vi "AeroQuadConfigurator.vi"() -> ()   [LabVIEW 2010] (continued)
              n282 = call "NextState.vi"("Data"=w567, "State"="Read", "Queue In"=w568) -> ()  [unwired: 7 in, 2 out]
            }
          }
          n283 = case shown="Error" w562 {
            selector: w562 -> [w578 w585]
            tunnel: [w578 w583] -> w563
            tunnel: w561 -> [_ _]
            tunnel: w558 -> [_ w588]
            tunnel: [TRUE ("Time has Elapsed") w587] -> w555
            tunnel: w556 -> [_ w584]
            tunnel: w550 -> [w576 _]
            tunnel: w553 -> [w574 _]
            frame No Error {
              n284 = Fract/Exp String To Number(string=w576) -> (number=w573:dbl)  [unwired: 3 in, 1 out]
              n285 = Greater Or Equal?(x=w573, y=w574) -> (x >= y?=w575:bool)
              n286 = case shown="False" w575 {
                tunnel: w573 -> [w580 _]
                tunnel: w574 -> [w579 _]
                frame False {
                  n287 = Format Into String(format string="To use all the features of this version of the Configurator, you must use Flight Software v.%.1f or greater.  The current detected Flight Software version is v.%.1f.", w579, w580) -> (resulting string=w582:string)  [unwired: 2 in, 1 out]
                  n288 = One Button Dialog(message=w582) -> ()  [unwired: 1 in, 1 out]
                }
                frame True {
                }
              }
            }
            frame Error {
              n289 = call "Elapsed Time"("Time Target (s)"=w588, "Reset"=w584) -> ("Time has Elapsed"=w587:bool, "error out"=w586:errorcluster)  [unwired: 10 in, 6 out]
              n290 = Select(t=w585, s=w587, f=w586) -> (s? t:f=w583:errorcluster)
            }
          }
        }
        n291 = Bundle By Name(cluster=w545, "Error"=w539) -> (w544:T2)
      }
      frame "Connect" {
        n292 = Unbundle By Name(w596) -> ("Logger"=w591:bool, "DebugLogger"=w595:refnum<queue>)  [unwired: 1 out]
        n293 = Unbundle By Name(w596) -> ("COM Port"=w606:refnum<visa-resource-name>, "StopTelem"=w594:string, "Version"=w593:string)
        n294 = VISA Write(VISA resource name=w606, write buffer=w594) -> (VISA resource name out=w603:refnum<visa-resource-name>, error out=w602:errorcluster)  [unwired: 1 in, 1 out]
        n295 = call "Time Delay8"("error in (no error)"=w602) -> ("error out"=w601:errorcluster)  [unwired: 10 in]
        n296 = VISA Flush I/O Buffer(VISA resource name=w603, error in (no error)=w601) -> (VISA resource name out=w604:refnum<visa-resource-name>, error out=w605:errorcluster)  [unwired: 1 in]
        n297 = VISA Write(VISA resource name=w604, write buffer=w593, error in (no error)=w605) -> (VISA resource name out=w612:refnum<visa-resource-name>, error out=w611:errorcluster)  [unwired: 1 out]
        n298 = VISA Read(VISA resource name=w612, byte count=u32 1024, error in (no error)=w611) -> (VISA resource name out=w609:refnum<visa-resource-name>, read buffer=w592:string, error out=w610:errorcluster)  [unwired: 1 out]
        n299 = case shown="True" w591 {
          selector: w591 -> [_ w625]
          tunnel: w595 -> [w623 w633]
          tunnel: w594 -> [_ w632]
          tunnel: w593 -> [_ w629]
          tunnel: w592 -> [_ w626]
          tunnel: [_ w625] -> w590
          tunnel: [w623 w624] -> w589
          frame False {
          }
          frame True {
            n300 = call "NextState.vi"("Data"=w632, "State"="Write", "Queue In"=w633) -> ("Queue Out"=w630:refnum<queue>)  [unwired: 7 in, 1 out]
            n301 = call "NextState.vi"("Data"=w629, "State"="Write", "Queue In"=w630) -> ("Queue Out"=w627:refnum<queue>)  [unwired: 7 in, 1 out]
            n302 = call "NextState.vi"("Data"=w626, "State"="Read", "Queue In"=w627) -> ("Queue Out"=w624:refnum<queue>)  [unwired: 7 in, 1 out]
          }
        }
        n303 = Decimal String To Number(string=w592) -> (number=w607:i32)  [unwired: 2 in, 1 out]
        n304 = local read "*Timeout (sec)"() -> (w598:dbl)
        n305 = for {
          N: w607 -> [_]
          tunnel: w609 -> [w647]
          shift-right: [w644] -> w619
          shift-left: w610 -> [w645]
          tunnel: [w641] -> w617 mode=indexing
          tunnel: [w640] -> w616 mode=indexing
          tunnel: [w639] -> w613 mode=indexing
          tunnel: [w638] -> w600
          tunnel: w590 -> [w637]
          tunnel: w589 -> [w636]
          n306 = VISA Read(VISA resource name=w647, byte count=u32 1024, error in (no error)=w645) -> (VISA resource name out=w638:refnum<visa-resource-name>, read buffer=w635:string, error out=w644:errorcluster)  [unwired: 1 out]
          n307 = Match Pattern(string=w635, regular expression=":") -> (before substring=w641:string, after substring=w642:string)  [unwired: 1 in, 2 out]
          n308 = case shown="True" w637 {
            tunnel: w636 -> [_ w650]
            tunnel: w635 -> [_ w648]
            frame False {
            }
            frame True {
              n309 = call "NextState.vi"("Data"=w648, "State"="Read", "Queue In"=w650) -> ()  [unwired: 7 in, 2 out]
            }
          }
          n310 = call <vilib>:"Trim Whitespace.vi"("string"=w642) -> ("trimmed string"=w640:string)  [unwired: 1 in]
          n311 = Build Array(w641, w640) -> (w639:string[])
        }
        n312 = Multiply(x=w598, y=1000.0) -> (x*y=w599:dbl)
        n313 = property class="Instr"(reference=w600, "General Settings:Timeout Value"=w599) -> ()  [unwired: 1 in, 2 out]
        n314 = Unbundle By Name(w619) -> ("status"=w618:bool)
        n315 = property on="Sensors" class="Tbl (strict)"("Row Headers[]"=w617) -> ()  [unwired: 2 in, 2 out]
        n316 = Build Array(w616) -> (w615:string[][])
        n317 = Not(x=w618) -> (.not. x?=w620:bool)
        n318 = case shown="True" w620 {
          tunnel: w621 -> [_ w657]
          frame False {
          }
          frame True {
            n319 = call "NextStates.vi"("States"=string[] ["Update Parameters", "Unlock Controls", "Save Comm Controls", "Lock Comm Controls", "Unlock User Controls"], "Queue In"=w657) -> ("Queue Out"=w653:refnum<queue>)  [unwired: 8 in, 1 out]
            n320 = call "NextState.vi"("Data"="Connected to the AeroQuad!", "State"="Status", "Queue In"=w653) -> ("Queue Out"=w652:refnum<queue>)  [unwired: 7 in, 1 out]
            n321 = call <vilib>:"Beep.vi"() -> ()  [unwired: 12 in]
            n322 = call "NextState.vi"("State"="Load SubPanel", "Queue In"=w652) -> ()  [unwired: 8 in, 2 out]
          }
        }
        n323 = Transpose 2D Array(2D array=w615) -> (transposed array=→"Sensors":string[][])
        n324 = Bundle By Name(cluster=w596, "Config"=w613, "Connected"=w620, "Error"=w619) -> (w622:T2)
      }
      frame "Request Telemetry", "Send Command" {
        # "In a telemetry query, a command will be sent\nfirst, then a telemetry request."
        n325 = Unbundle By Name(w669) -> ("Logger"=w658:bool, "DebugLogger"=w659:refnum<queue>, "oldTelem"=w660:string, "Connected"=w666:bool, "COM Port"=w670:refnum<visa-resource-name>)
        n326 = case shown="True" w666 {
          tunnel: w670 -> [_ w679]
          tunnel: w667 -> [_ w681]
          tunnel: [_ w680] -> w665
          tunnel: w664 -> [w671 _]
          tunnel: w663 -> [w673 _]
          tunnel: [_ w675] -> w662
          tunnel: [_ w678] -> w661
          tunnel: w660 -> [_ w678]
          tunnel: w659 -> [_ w676]
          tunnel: w658 -> [_ w677]
          frame False {
            n327 = Flush Queue(queue=w671) -> (queue out=w672:refnum<queue>)  [unwired: 1 in, 2 out]
            n328 = case shown="\"Send Command\"" w673 {
              tunnel: w672 -> [_ _]
              frame Default {
              }
              frame "Send Command" {
                n329 = One Button Dialog(message="The AeroQuad is not connected to the Configurator!\nErroneous messages may appear.") -> ()  [unwired: 1 in, 1 out]
              }
            }
          }
          frame True {
            n330 = Variant To Data(Variant=w681, type="") -> (data=w675:string)  [unwired: 1 in, 1 out]
            n331 = VISA Write(VISA resource name=w679, write buffer=w675) -> (error out=w680:errorcluster)  [unwired: 1 in, 2 out]
            n332 = case shown="True" w677 {
              tunnel: w676 -> [_ w685]
              tunnel: w675 -> [_ w683]
              frame False {
              }
              frame True {
                n333 = call "NextState.vi"("Data"=w683, "State"="Write", "Queue In"=w685) -> ()  [unwired: 7 in, 2 out]
              }
            }
          }
        }
        n334 = Bundle By Name(cluster=w669, "oldCmd"=w661, "oldTelem"=w662, "Error"=w665) -> (w668:T2)
      }
      frame "Clear Serial Comm" {
        n335 = Unbundle By Name(w692) -> ("Logger"=w687:bool, "DebugLogger"=w686:refnum<queue>, "Connected"=w690:bool, "COM Port"=w693:refnum<visa-resource-name>, "StopTelem"=w688:string)
        n336 = case shown="True" w690 {
          tunnel: w693 -> [_ w704]
          tunnel: [_ w701] -> w689
          tunnel: w688 -> [_ w694]
          tunnel: w687 -> [_ w696]
          tunnel: w686 -> [_ w695]
          frame False {
          }
          frame True {
            n337 = case shown="True" w696 {
              tunnel: w695 -> [_ w709]
              tunnel: w694 -> [_ w708]
              tunnel: w694 -> [_ w705]
              frame False {
              }
              frame True {
                w706 = "Write" ("State")
                n338 = call "NextState.vi"("Data"=w708, "State"=w706, "Queue In"=w709) -> ("Queue Out"=w707:refnum<queue>)  [unwired: 7 in, 1 out]
                n339 = disable-structure shown="Disabled" {
                  disable-tunnel: w707 -> [w712 _]
                  disable-tunnel: w706 -> [w711 _]
                  disable-tunnel: w705 -> [w710 _]
                  frame Disabled {
                    n340 = call "NextState.vi"("Data"=w710, "State"=w711, "Queue In"=w712) -> ()  [unwired: 7 in, 2 out]
                  }
                  frame Enabled {
                  }
                }
              }
            }
            n341 = VISA Write(VISA resource name=w704, write buffer=w694) -> (VISA resource name out=w699:refnum<visa-resource-name>, error out=w702:errorcluster)  [unwired: 1 in, 1 out]
            n342 = call "Time Delay3"("error in (no error)"=w702, "Delay Time (s)"=0.25) -> ("error out"=w698:errorcluster)  [unwired: 9 in]
            n343 = VISA Flush I/O Buffer(VISA resource name=w699, error in (no error)=w698) -> (VISA resource name out=w700:refnum<visa-resource-name>, error out=w697:errorcluster)  [unwired: 1 in]
            n344 = disable-structure shown="Enabled" {
              disable-tunnel: [w720 w721] -> w701
              disable-tunnel: w694 -> [w719 _]
              disable-tunnel: w700 -> [w714 _]
              disable-tunnel: w697 -> [w713 w721]
              frame Disabled {
                n345 = VISA Write(VISA resource name=w714, write buffer=w719, error in (no error)=w713) -> (VISA resource name out=w715:refnum<visa-resource-name>, error out=w717:errorcluster)  [unwired: 1 out]
                n346 = call "Time Delay5"("error in (no error)"=w717, "Delay Time (s)"=0.25) -> ("error out"=w716:errorcluster)  [unwired: 9 in]
                n347 = VISA Flush I/O Buffer(VISA resource name=w715, error in (no error)=w716) -> (error out=w720:errorcluster)  [unwired: 1 in, 1 out]
              }
              frame Enabled {
              }
            }
          }
        }
        n348 = Bundle By Name(cluster=w692, "Error"=w689) -> (w691:T2)
      }
      frame "Reconnect" {
        n349 = in-place {
          in-place-border: [w732] -> w724
          n350 = in-place-cluster #3(w727) -> ("Error"=w734:errorcluster)
          n351 = call "ReconnectDialog.vi"("error in"=w734) -> ("error out"=w733:errorcluster, "AbortConnection"=w732:bool)  [unwired: 9 in]
          n352 = in-place-cluster #3("Error"=w733) -> (w726:T2)
        }
        n353 = case shown="False" w724 {
          tunnel: w725 -> [w729 w731]
          tunnel: [w729 w731] -> w723
          tunnel: ["Open Port" "Unlock User Controls"] -> w722
          frame False {
          }
          frame True {
          }
        }
        n354 = call "NextState.vi"("State"=w722, "Queue In"=w723) -> ()  [unwired: 8 in, 2 out]
      }
      frame "Disconnect" {
        n355 = property on="Load SubPanel" class="Ring (strict)"() -> ("Strings []"=w744:string[], "Value"=w745:i32)  [unwired: 2 in, 2 out]
        n356 = Unbundle By Name(w758) -> ("ConnType"=w741:string, "ModemQueue"=w736:refnum<queue>, "COM Port"=w748:refnum<visa-resource-name>, "StopTelem"=w746:string)
        n357 = Index Array(array=w744, index=w745) -> (element=w743:string)
        n358 = call "NextState.vi"("State"="Lock Controls", "Queue In"=w754) -> ("Queue Out"=w752:refnum<queue>)  [unwired: 8 in, 1 out]
        n359 = VISA Write(VISA resource name=w748, write buffer=w746) -> (VISA resource name out=w747:refnum<visa-resource-name>)  [unwired: 1 in, 2 out]
        n360 = VISA Close(VISA resource name=w747) -> ()  [unwired: 1 in, 1 out]
        n361 = call "PriorityState.vi"("Data"="Disconnected from AeroQuad", "State"="Status", "Queue In"=w752) -> ("Queue Out"=w751:refnum<queue>)  [unwired: 7 in, 1 out]
        n362 = Equal?(x="Modem Telemetry Initialize", y=w741) -> (x = y?=w738:bool)
        n363 = Equal?(x="Waypoint Configuration", y=w743) -> (x = y?=w739:bool)
        n364 = Compound Arithmetic op=AND(w739, w738) -> (w737:bool)
        n365 = call "NextState.vi"("State"="Unlock Comm Controls", "Queue In"=w751) -> ("Queue Out"=w735:refnum<queue>)  [unwired: 8 in, 1 out]
        n366 = case shown="True" w737 {
          tunnel: w736 -> [_ w768]
          tunnel: w735 -> [w760 w770]
          frame False {
            n367 = call "NextState.vi"("State"="Unlock User Controls", "Queue In"=w760) -> ()  [unwired: 8 in, 2 out]
          }
          frame True {
            n368 = Flush Queue(queue=w768) -> (queue out=w767:refnum<queue>)  [unwired: 1 in, 2 out]
            n369 = Enqueue Element(queue=w767, element="***Disconnect***") -> (error out=w766:errorcluster)  [unwired: 2 in, 2 out]
            n370 = call "NextState.vi"("Error In"=w766, "State"="Lock User Controls", "Queue In"=w770) -> ("Queue Out"=w765:refnum<queue>)  [unwired: 7 in, 1 out]
            n371 = call "NextState.vi"("Data"="Disconnected from AeroQuad" ("State"), "State"="Status", "Queue In"=w765) -> ("Queue Out"=w762:refnum<queue>)  [unwired: 7 in, 1 out]
            n372 = call "NextState.vi"("State"="Clear Queue", "Queue In"=w762) -> ()  [unwired: 8 in, 2 out]
          }
        }
        n373 = Bundle By Name(cluster=w758, "Connected"=FALSE) -> (w757:T2)
      }
      frame "Update Timeout" {
        n374 = Unbundle By Name(w772) -> ("COM Port"=w776:refnum<visa-resource-name>)
        n375 = Variant To Data(Variant=w775, type=u32 0 ("General Settings:Timeout Value")) -> (data=w773:u32)  [unwired: 1 in, 1 out]
        n376 = property class="Instr"(reference=w776, "Timeout"=w773) -> ()  [unwired: 1 in, 2 out]
      }
      frame "Default Timeout" {
        n377 = Unbundle By Name(w781) -> ("COM Port"=w782:refnum<visa-resource-name>)
        n378 = local read "*Timeout (sec)"() -> (w778:dbl)
        n379 = Compound Arithmetic op=MULTIPLY(w778, 1000.0 ("value")) -> (w780:dbl)
        n380 = To Unsigned Long Integer(number=w780) -> (unsigned 32bit integer=w777:u32)
        n381 = property class="Instr"(reference=w782, "Timeout"=w777) -> ()  [unwired: 1 in, 2 out]
      }
      frame "Connection Type" {
        n382 = Variant To Data(Variant=w785, type="") -> (data=w783:string)  [unwired: 1 in, 1 out]
        n383 = case shown="\"Modem\"" w783 {
          tunnel: w789 -> [w791 w797]
          tunnel: ["Modem Telemetry Initialize" "Check Connection"] -> w786
          frame "Modem" {
            w795 = 3 items=["Initial Setup", "3-D View", "Vehicle Status", "Waypoint Configuration", "Motor Commands", "Serial Monitor", "Vehicle Attitude", "Sensor Data", "Transmitter Data"] ("Load SubPanel")
            n384 = call "NextState.vi"("State"="Lock User Controls", "Queue In"=w791) -> ("Queue Out"=w790:refnum<queue>)  [unwired: 8 in, 1 out]
            n385 = local write "Load SubPanel"(w795) -> ()
            n386 = local write "*Baud Rate"("1200" ("*Baud Rate")) -> ()
            n387 = call "NextState.vi"("State"="Load SubPanel", "Queue In"=w790) -> ()  [unwired: 8 in, 2 out]
          }
          frame "USB/XBee", Default {
            n388 = call "NextState.vi"("State"="Unlock User Controls", "Queue In"=w797) -> ()  [unwired: 8 in, 2 out]
            n389 = property on="Load SubPanel" class="Ring (strict)"("DisabledEnum"=T3."Enabled" ("Disabled")) -> ()  [unwired: 2 in, 2 out]
          }
        }
        n390 = Bundle By Name(cluster=w788, "ConnType"=w786) -> (w787:T2)
      }
      frame "Modem Telemetry Initialize" {
        # "Modem queue initialized in \"Load SubPanels\" state for convenience."
        n391 = Unbundle By Name(w807) -> ("ModemQueue"=w803:refnum<queue>)
        n392 = call "NextState.vi"("State"="Unlock Controls", "Queue In"=w815) -> ("Queue Out"=w811:refnum<queue>)  [unwired: 8 in, 1 out]
        n393 = Lossy Enqueue Element(queue=w803, element="Move Slider Modem" ("State")) -> (queue out=w801:refnum<queue>)  [unwired: 1 in, 3 out]
        n394 = call "NextState.vi"("State"="Lock User Controls", "Queue In"=w811) -> ("Queue Out"=w810:refnum<queue>)  [unwired: 8 in, 1 out]
        n395 = Lossy Enqueue Element(queue=w801, element="Fresh Data") -> ()  [unwired: 1 in, 4 out]
        n396 = Bundle By Name(cluster=w807, "Stale"=0) -> (w806:T2)
        n397 = call "NextState.vi"("State"="Lock Comm Controls", "Queue In"=w810) -> ("Queue Out"=w809:refnum<queue>)  [unwired: 8 in, 1 out]
        n398 = call "NextState.vi"("State"="Modem Telemetry Read", "Queue In"=w809) -> ()  [unwired: 8 in, 2 out]
      }
      frame "Modem Telemetry Read" {
        n399 = Unbundle By Name(w819) -> ("Logger"=w817:bool, "DebugLogger"=w816:refnum<queue>, "ModemQueue"=w828:refnum<queue>, "COM Port"=w830:refnum<visa-resource-name>, "Stale"=w821:i32)
        n400 = VISA Read(VISA resource name=w830, byte count=u32 16) -> (read buffer=w827:string, error out=w826:errorcluster)  [unwired: 1 in, 2 out]
        n401 = case shown="No Error" w826 {
          selector: w826 -> [w840 _]
          tunnel: w828 -> [w841 w854]
          tunnel: w827 -> [w831 _]
          tunnel: [w835 w858] -> w823
          tunnel: w825 -> [w837 w859]
          tunnel: "No data from modem, retrying..." -> [w839 w857]
          tunnel: w821 -> [_ w853]
          tunnel: [_ w852] -> w820
          tunnel: w817 -> [w833 _]
          tunnel: w816 -> [w832 _]
          frame No Error {
            n402 = local read "Status"() -> (w838:string)
            n403 = Lossy Enqueue Element(queue=w841, element=w831, error in (no error)=w840) -> (queue out=w834:refnum<queue>)  [unwired: 3 out]
            n404 = Equal?(x=w839, y=w838) -> (x = y?=w836:bool)
            n405 = case shown="True" w836 {
              tunnel: w837 -> [w845 w851]
              tunnel: [w845 w850] -> w835
              tunnel: w834 -> [_ w847]
              frame False {
              }
              frame True {
                n406 = call "NextState.vi"("Data"="Receiving data from the modem...", "State"="Status", "Queue In"=w851) -> ("Queue Out"=w850:refnum<queue>)  [unwired: 7 in, 1 out]
                n407 = Lossy Enqueue Element(queue=w847, element="Fresh Data") -> ()  [unwired: 1 in, 4 out]
              }
            }
            n408 = case shown="True" w833 {
              tunnel: w832 -> [_ w844]
              tunnel: w831 -> [_ w842]
              frame False {
              }
              frame True {
                n409 = call "NextState.vi"("Data"=w842, "State"="Read", "Queue In"=w844) -> ()  [unwired: 7 in, 2 out]
              }
            }
          }
          frame Error {
            n410 = Greater?(x=w853, y=10) -> (0:w855:bool)
            n411 = Increment(x=w853) -> (x+1=w852:i32)
            n412 = case shown="True" w855 {
              tunnel: w854 -> [_ w862]
              frame False {
              }
              frame True {
                n413 = Lossy Enqueue Element(queue=w862, element="Stale Data") -> ()  [unwired: 1 in, 4 out]
              }
            }
            n414 = call "NextState.vi"("Data"=w857, "State"="Status", "Queue In"=w859) -> ("Queue Out"=w858:refnum<queue>)  [unwired: 7 in, 1 out]
          }
        }
        n415 = Bundle By Name(cluster=w819, "Stale"=w820) -> (w818:T2)
        n416 = call "NextState.vi"("State"="Modem Telemetry Read", "Queue In"=w823) -> ()  [unwired: 8 in, 2 out]
      }
      frame "Communication Log" {
        n417 = Variant To Data(Variant=w871, type="") -> (data=w869:string)  [unwired: 1 in, 1 out]
        n418 = Unbundle By Name(w865) -> ("DebugLogger"=w864:refnum<queue>)
        n419 = case shown="\"Clean Up\"" w869 {
          tunnel: [_ _ TRUE] -> w867
          tunnel: w866 -> [w877 _ _]
          tunnel: w864 -> [w873 w878 _]
          tunnel: [w872 _ w884] -> w863
          frame "Close", Default {
            n420 = call "NextState.vi"("State"="Close", "Queue In"=w873) -> ("Queue Out"=w872:refnum<queue>)  [unwired: 8 in, 1 out]
            n421 = call "NextState.vi"("Data"="Clean Up" ("State"), "State"="Communication Log", "Queue In"=w877) -> ()  [unwired: 7 in, 2 out]
          }
          frame "Clean Up" {
            n422 = Current VI's Menubar() -> (w883:refnum<k9>)
            n423 = Set Menu Item Info(6:FALSE ("checked"), 7:"Communication Log" ("item tag"), 11:w883) -> ()  [unwired: 4 in, 2 out]
            n424 = call "NextState.vi"("State"="Close", "Queue In"=w878) -> ("Queue Out"=w879:refnum<queue>)  [unwired: 8 in, 1 out]
            n425 = Release Queue(queue=w879) -> ()  [unwired: 2 in, 3 out]
          }
          frame "Open" {
            n426 = call "InitState.vi"("Name"="DebugLog") -> ("Error Out"=w885:errorcluster, "Queue Out"=w884:refnum<queue>)  [unwired: 8 in]
            n427 = property class="App"(error in=w885) -> ("App.Kind"=w895:T8)  [unwired: 1 in, 2 out]
            n428 = case shown="\"Development System\"" w895 {
              tunnel: [w898 w901] -> w893
              tunnel: path "Support/DebugLogger.vi" ("Output Path") -> [w897 w902]
              frame "Run Time System", Default {
                n429 = Current VI's Path() -> (path=w900:path)
                n430 = Strip Path(path=w900) -> (stripped path=w899:path)  [unwired: 1 out]
                n431 = Build Path(base path=w899, name or relative path=w897) -> (appended path=w898:path)
              }
              frame "Development System" {
                n432 = call <userlib>:"Current VIs Parent Directory__ogtk.vi"("Relative path (.)"=w902) -> ("Parent Directory (+ Relative)"=w901:path)  [unwired: 4 in]
              }
            }
            n433 = Open VI Reference(vi path=w893) -> (vi reference=w892:refnum<vi>)  [unwired: 5 in, 1 out]
            n434 = invoke class="VI" method="Run VI"(reference=w892, "Wait until done"=FALSE ("Wait Until Done"), "Auto Dispose Ref"=TRUE ("Auto Dispose Reference")) -> (reference out=w889:refnum<vi>)  [unwired: 2 in, 4 out]
            n435 = invoke class="VI" method="FP.Open"(reference=w889, "Activate"=TRUE ("Activate?"), "State"=T5."Standard") -> ()  [unwired: 2 in, 5 out]
          }
        }
        n436 = Bundle By Name(cluster=w865, "DebugLogger"=w863, "Logger"=w867) -> (w868:T2)
      }
      frame "--- Parameters ---" {
      }
      frame "Parameter Check" {
        # "Validate data in text table."
        n437 = local read "Parameter Type"() -> (w910:i32)
        n438 = Unbundle By Name(w917) -> ("Parameters"=w913:string[][][])
        n439 = Index Array(array=w913, index (dim 0)=w910, index (dim 2)=1 ("disabled index (col)")) -> (element=w915:string[])  [unwired: 1 in]
        n440 = Index Array(array="Parameter Check", index (col)=0 ("disabled index (col)")) -> (element=w908:string[])  [unwired: 1 in]
        n441 = Split 1D Array(array=w915, index=2) -> (second subarray=w912:string[])  [unwired: 1 out]
        n442 = for {
          tunnel: w912 -> [w919] mode=indexing
          tunnel: [w918] -> w906 mode=indexing
          tunnel: w908 -> [w924] mode=indexing
          n443 = call <vilib>:"Trim Whitespace.vi"("string"=w924) -> ("trimmed string"=w923:string)  [unwired: 1 in]
          n444 = Search and Replace String(replace all?=TRUE ("replace all? (F)"), input string=w923, search string=",", replace string="." ("replace string (\"\")")) -> (result string=w928:string)  [unwired: 4 in, 3 out]
          n445 = Fract/Exp String To Number(use system decimal point (T)=FALSE, string=w928) -> (offset past number=w922:i32, number=w930:dbl)  [unwired: 2 in]
          n446 = Greater Than 0?(x=w922) -> (x > 0?=w921:bool)
          n447 = Format Value(format string="%#g", value (0)=w930) -> (output string=w920:string)  [unwired: 1 in]
          n448 = Select(t=w920, s=w921, f=w919) -> (s? t:f=w918:string)
        }
        n449 = Replace Array Subset(array="Parameter Check", new element=w906, index (col)=0 ("disabled index (col)")) -> (w909:string[][])  [unwired: 1 in]
        n450 = local write "Parameter Check"(w909) -> ()
        n451 = property on="Parameter Check" class="Tbl (strict)"("Selection Start"=T6 {"Row"=10, "Column"=10} ("Selection Size")) -> ()  [unwired: 2 in, 2 out]
      }
      frame "Parameter Type" {
        # "Load paramater values into table"
        # "Load paramater names into table"
        n452 = Unbundle By Name(w949) -> ("Parameters"=w948:string[][][])
        n453 = Index Array(array=w948, index (dim 0)="Parameter Type", index (dim 2)=1 ("disabled index (col)")) -> (element=w943:string[])  [unwired: 1 in]
        n454 = Split 1D Array(array=w943, index=2) -> (second subarray=w937:string[])  [unwired: 1 out]
        n455 = Index Array(array=w948, index (dim 0)="Parameter Type", index (dim 2)=0 ("disabled index (col)")) -> (element=w941:string[])  [unwired: 1 in]
        n456 = Split 1D Array(array=w941, index=2) -> (second subarray=w933:string[])  [unwired: 1 out]
        n457 = Search 1D Array(1D array=w933, element="") -> (index of element=w935:i32)  [unwired: 1 in]
        n458 = case shown="..0" w935 {
          selector: w935 -> [_ w952]
          tunnel: [w951 w952] -> w934
          tunnel: w933 -> [w950 _]
          frame ..0 {
            n459 = Array Size(array=w950) -> (size(s)=w951:i32)
          }
          frame Default {
          }
        }
        n460 = property on="Parameter Check" class="Tbl (strict)"("Selection Start"=T7 {"Row"=10, "Column"=10} ("Index Values"), "Row Headers[]"=w933) -> ()  [unwired: 2 in, 2 out]
        n461 = Split 1D Array(array=w937, index=w934) -> (first subarray=w938:string[])  [unwired: 1 out]
        n462 = Build Array(w938) -> (w945:string[][])
        n463 = Transpose 2D Array(2D array=w945) -> (transposed array=w944:string[][])
        n464 = local write "Parameter Check"(w944) -> ()
      }
      frame "Update Parameters" {
        n465 = Unbundle By Name(w969) -> ("Parameters"=w967:string[][][], "COM Port"=w966:refnum<visa-resource-name>, "Error"=w958:errorcluster, "DebugLogger"=w954:refnum<queue>, "Logger"=w953:bool)
        n466 = call "Time Delay7"("error in (no error)"=w958) -> ("error out"=w959:errorcluster)  [unwired: 10 in]
        n467 = for {
          tunnel: w967 -> [w983] mode=indexing
          tunnel: w966 -> [w986]
          shift-right: [w978] -> w965
          shift-left: w959 -> [w984]
          shift-right: [w976] -> w964
          shift-left: string[][] [] -> [w977]
          shift-right: [w975] -> w955
          shift-left: string[][][] [] ("Parameters") -> [w974]
          tunnel: w954 -> [w972]
          tunnel: w953 -> [w973]
          n468 = Index Array(array=w983, index (col)=0 ("disabled index (col)")) -> (element=w990:string[])  [unwired: 1 in]
          n469 = Search 1D Array(1D array=w990, element="Telemetry") -> (index of element=w988:i32)  [unwired: 1 in]
          n470 = Index Array(array=w983, index (row)=w988, index (col)=1 ("disabled index (col)")) -> (element=w970:string)
          n471 = VISA Write(VISA resource name=w986, write buffer=w970, error in (no error)=w984) -> (VISA resource name out=w980:refnum<visa-resource-name>, error out=w982:errorcluster)  [unwired: 1 out]
          n472 = call "Time Delay2"("error in (no error)"=w982) -> ("error out"=w981:errorcluster)  [unwired: 10 in]
          n473 = VISA Read(VISA resource name=w980, byte count=u32 1024, error in (no error)=w981) -> (read buffer=w971:string, error out=w979:errorcluster)  [unwired: 2 out]
          n474 = case shown="True" w973 {
            tunnel: w972 -> [_ w997]
            tunnel: w971 -> [_ w994]
            tunnel: w970 -> [_ w992]
            frame False {
            }
            frame True {
              n475 = call "NextState.vi"("Data"=w992, "State"="Write", "Queue In"=w997) -> ("Queue Out"=w996:refnum<queue>)  [unwired: 7 in, 1 out]
              n476 = call "NextState.vi"("Data"=w994, "State"="Read", "Queue In"=w996) -> ()  [unwired: 7 in, 2 out]
            }
          }
          n477 = case shown="No Error" w979 {
            selector: w979 -> [w1004 w1025]
            tunnel: w983 -> [w1008 _]
            tunnel: [w999 w1024] -> w975
            tunnel: w971 -> [w1005 _]
            tunnel: [w1004 w1025] -> w978
            tunnel: w977 -> [w1003 w1023]
            tunnel: [w1001 w1023] -> w976
            tunnel: w974 -> [w998 w1024]
            frame No Error {
              n478 = call "RemoveTrailingComma.vi"("Input String"=w1005) -> ("Output String"=w1006:string)  [unwired: 8 in]
              n479 = Spreadsheet String To Array(delimiter (Tab)=",", format string="%s", spreadsheet string=w1006, array type (2D Dbl)=string[] []) -> (array=w1007:string[])
              n480 = for {
                shift-right: [w1021] -> w1000
                shift-left: w1008 -> [w1022]
                tunnel: w1007 -> [w1013] mode=indexing
                tunnel: [w1012] -> w1002 mode=indexing
                i -> [w1018]
                n481 = Fract/Exp String To Number(use system decimal point (T)=FALSE, string=w1013) -> (number=w1015:dbl)  [unwired: 2 in, 1 out]
                n482 = Format Value(format string="%#g", value (0)=w1015) -> (output string=w1012:string)  [unwired: 1 in]
                n483 = Compound Arithmetic op=ADD(2 ("disabled index (row)"), w1018) -> (w1017:i32)
                n484 = Replace Array Subset(array=w1022, new element=w1012, index (row)=w1017, index (col)=1 ("disabled index (col)")) -> (w1021:string[][])
              }
              n485 = Build Array (concatenate)(w1003, w1002) -> (w1001:string[][])
              n486 = Build Array (concatenate)(w998, w1000) -> (w999:string[][][])
            }
            frame Error {
              # "Don't error out if parameter not found."
            }
          }
        }
        n487 = local read "Parameter Type"() -> (w963:i32)
        n488 = Bundle By Name(cluster=w969, "Parameters"=w955, "Error"=w965) -> (w968:T2)
        n489 = Index Array(array=w964, index (row)=w963) -> (element=w962:string[])  [unwired: 1 in]
        n490 = Build Array(w962) -> (w961:string[][])
        n491 = Transpose 2D Array(2D array=w961) -> (transposed array=w960:string[][])
        n492 = local write "Parameter Check"(w960) -> ()
      }
      frame "Update Parameter" {
        n493 = Unbundle By Name(w1056) -> ("Parameters"=w1037:string[][][], "COM Port"=w1054:refnum<visa-resource-name>, "Error"=w1053:errorcluster, "DebugLogger"=w1028:refnum<queue>, "Logger"=w1029:bool)
        n494 = local read "Parameter Type"() -> (w1036:i32)
        n495 = Index Array(array=w1037, index (dim 0)=w1036) -> (element=w1038:string[][])  [unwired: 2 in]
        n496 = Index Array(array=w1038, index (col)=0 ("disabled index (col)")) -> (element=w1050:string[])  [unwired: 1 in]
        n497 = Search 1D Array(1D array=w1050, element="Telemetry") -> (index of element=w1048:i32)  [unwired: 1 in]
        n498 = Index Array(array=w1038, index (row)=w1048, index (col)=1 ("disabled index (col)")) -> (element=w1027:string)
        n499 = VISA Write(VISA resource name=w1054, write buffer=w1027, error in (no error)=w1053) -> (VISA resource name out=w1040:refnum<visa-resource-name>, error out=w1042:errorcluster)  [unwired: 1 out]
        n500 = call "Time Delay6"("error in (no error)"=w1042) -> ("error out"=w1041:errorcluster)  [unwired: 10 in]
        n501 = VISA Read(VISA resource name=w1040, byte count=u32 1024, error in (no error)=w1041) -> (read buffer=w1026:string, error out=w1052:errorcluster)  [unwired: 2 out]
        n502 = case shown="True" w1029 {
          tunnel: w1028 -> [_ w1062]
          tunnel: w1027 -> [_ w1060]
          tunnel: w1026 -> [_ w1057]
          frame False {
          }
          frame True {
            n503 = call "NextState.vi"("Data"=w1060, "State"="Write", "Queue In"=w1062) -> ("Queue Out"=w1058:refnum<queue>)  [unwired: 7 in, 1 out]
            n504 = call "NextState.vi"("Data"=w1057, "State"="Write", "Queue In"=w1058) -> ()  [unwired: 7 in, 2 out]
          }
        }
        n505 = call "RemoveTrailingComma.vi"("Input String"=w1026) -> ("Output String"=w1030:string)  [unwired: 8 in]
        n506 = Spreadsheet String To Array(delimiter (Tab)=",", format string="%s", spreadsheet string=w1030, array type (2D Dbl)=string[] []) -> (array=w1039:string[])
        n507 = for {
          shift-right: [w1072] -> w1034
          shift-left: w1038 -> [w1073]
          tunnel: w1039 -> [w1064] mode=indexing
          tunnel: [w1063] -> w1033 mode=indexing
          i -> [w1069]
          n508 = Fract/Exp String To Number(use system decimal point (T)=FALSE, string=w1064) -> (number=w1066:dbl)  [unwired: 2 in, 1 out]
          n509 = Format Value(format string="%#g", value (0)=w1066) -> (output string=w1063:string)  [unwired: 1 in]
          n510 = Compound Arithmetic op=ADD(2 ("disabled index (row)"), w1069) -> (w1068:i32)
          n511 = Replace Array Subset(array=w1073, new element=w1063, index (row)=w1068, index (col)=1 ("disabled index (col)")) -> (w1072:string[][])
        }
        n512 = Build Array(w1033) -> (w1032:string[][])
        n513 = Transpose 2D Array(2D array=w1032) -> (transposed array=w1031:string[][])
        n514 = local write "Parameter Check"(w1031) -> ()
        n515 = Replace Array Subset(array=w1037, new element=w1034, index (dim 0)=w1036) -> (w1035:string[][][])  [unwired: 2 in]
        n516 = Bundle By Name(cluster=w1056, "Parameters"=w1035, "Error"=w1052) -> (w1055:T2)
      }
      frame "Easy Update" {
        # "Load SubPanel in case it was previously communicating"
        n517 = Variant To Data(Variant=w1079, type=w1078) -> (data=w1077:string)  [unwired: 1 in, 1 out]
        n518 = local read "Parameter Type"() -> (w1086:i32)
        n519 = Unbundle By Name(w1093) -> ("Parameters"=w1087:string[][][])
        n520 = call "NextState.vi"("State"="Load SubPanel", "Queue In"=w1074) -> ()  [unwired: 8 in, 2 out]
        n521 = call "RemoveTrailingComma.vi"("Input String"=w1077) -> ("Output String"=w1080:string)  [unwired: 8 in]
        n522 = Index Array(array=w1087, index (dim 0)=w1086) -> (element=w1076:string[][])  [unwired: 2 in]
        n523 = Spreadsheet String To Array(delimiter (Tab)=",", format string="%s", spreadsheet string=w1080, array type (2D Dbl)=string[] []) -> (array=w1088:string[])
        n524 = for {
          shift-right: [w1103] -> w1084
          shift-left: w1076 -> [w1104]
          tunnel: w1088 -> [w1095] mode=indexing
          tunnel: [w1094] -> w1083 mode=indexing
          i -> [w1100]
          n525 = Fract/Exp String To Number(use system decimal point (T)=FALSE, string=w1095) -> (number=w1097:dbl)  [unwired: 2 in, 1 out]
          n526 = Format Value(format string="%#g", value (0)=w1097) -> (output string=w1094:string)  [unwired: 1 in]
          n527 = Compound Arithmetic op=ADD(2 ("disabled index (row)"), w1100) -> (w1099:i32)
          n528 = Replace Array Subset(array=w1104, new element=w1094, index (row)=w1099, index (col)=1 ("disabled index (col)")) -> (w1103:string[][])
        }
        n529 = Build Array(w1083) -> (w1082:string[][])
        n530 = Transpose 2D Array(2D array=w1082) -> (transposed array=w1081:string[][])
        n531 = local write "Parameter Check"(w1081) -> ()
        n532 = Replace Array Subset(array=w1087, new element=w1084, index (dim 0)=w1086) -> (w1085:string[][][])  [unwired: 2 in]
        n533 = Bundle By Name(cluster=w1093, "Parameters"=w1085) -> (w1092:T2)
      }
      frame "Upload" {
        w1105 = T3."Disabled and Grayed Out" ("Disabled")
        n534 = Flush Queue(queue=w1107) -> (queue out=w1106:refnum<queue>)  [unwired: 1 in, 2 out]
        n535 = Unbundle By Name(w1150) -> ("Parameters"=w1125:string[][][])
        n536 = local read "Parameter Check"() -> (w1147:string[][])
        n537 = local read "Parameter Type"() -> (w1124:i32)
        n538 = call "NextState.vi"("Data"="Uploading to AeroQuad", "State"="Status", "Queue In"=w1106) -> ("Queue Out"=w1114:refnum<queue>)  [unwired: 7 in, 1 out]
        n539 = Index Array(array=w1147, index (col)=0 ("disabled index (col)")) -> (element=w1130:string[])  [unwired: 1 in]
        n540 = call "NextState.vi"("State"="Clear Serial Comm", "Queue In"=w1114) -> ("Queue Out"=w1110:refnum<queue>)  [unwired: 8 in, 1 out]
        n541 = Index Array(array=w1125, index (dim 0)=w1124, index (dim 2)=0 ("disabled index (row)")) -> (element=w1138:string[])  [unwired: 1 in]
        n542 = Array To Spreadsheet String(delimiter (Tab)=";", array=w1130, 3:"%s" ("format string")) -> (spreadsheet string=w1119:string)
        n543 = Search 1D Array(1D array=w1138, element="Command") -> (index of element=w1127:i32)  [unwired: 1 in]
        n544 = Match Pattern(string=w1119, regular expression=";;") -> (before substring=w1121:string)  [unwired: 4 out]
        n545 = Index Array(array=w1125, index (dim 0)=w1124, index (dim 1)=w1127, index (dim 2)=1 ("disabled index (col)")) -> (element=w1141:string)
        n546 = call "NextState.vi"("State"="Default Timeout", "Queue In"=w1110) -> ("Queue Out"=w1109:refnum<queue>)  [unwired: 8 in, 1 out]
        n547 = Match Pattern(string=w1121, regular expression="\r\n") -> (before substring=w1131:string)  [unwired: 4 out]
        n548 = Format Into String(format string="%s%s;", w1141, w1131) -> (resulting string=w1140:string)  [unwired: 2 in, 1 out]
        n549 = Array To Spreadsheet String(delimiter (Tab)=",", array=w1130, 3:"%s" ("format string")) -> (spreadsheet string=w1116:string)
        n550 = Search 1D Array(1D array=w1138, element="Telemetry") -> (index of element=w1123:i32)  [unwired: 1 in]
        n551 = call "NextState.vi"("Data"=w1140, "State"="Send Command", "Queue In"=w1109) -> ("Queue Out"=w1136:refnum<queue>)  [unwired: 7 in, 1 out]
        n552 = Index Array(array=w1125, index (dim 0)=w1124, index (dim 1)=w1123, index (dim 2)=1 ("disabled index (col)")) -> (element=w1118:string)
        n553 = Match Pattern(string=w1116, regular expression=",,") -> (before substring=w1117:string)  [unwired: 4 out]
        n554 = Match Pattern(string=w1117, regular expression="\r\n") -> (before substring=w1113:string)  [unwired: 4 out]
        n555 = call "NextState.vi"("Data"=w1118, "State"="Request Telemetry", "Queue In"=w1136) -> ("Queue Out"=w1135:refnum<queue>)  [unwired: 7 in, 1 out]
        n556 = call "NextState.vi"("Data"=w1113, "State"="Verify Upload", "Queue In"=w1135) -> ("Queue Out"=w1112:refnum<queue>)  [unwired: 7 in, 1 out]
        n557 = disable-structure shown="Disabled" {
          disable-tunnel: w1112 -> [w1154 _]
          frame Disabled {
            n558 = call "NextState.vi"("State"="Update Parameter", "Queue In"=w1154) -> ("Queue Out"=w1153:refnum<queue>)  [unwired: 8 in, 1 out]
            n559 = call "NextState.vi"("State"="Load SubPanel", "Queue In"=w1153) -> ()  [unwired: 8 in, 2 out]
          }
          frame Enabled {
          }
        }
        n560 = property on="Upload" class="Bool"("DisabledEnum"=w1105) -> ()  [unwired: 2 in, 2 out]
        n561 = property on="Parameter Type" class="Ring (strict)"("DisabledEnum"=w1105) -> ()  [unwired: 2 in, 2 out]
      }
      frame "Update Tool Tip" {
        n562 = Unbundle By Name(w1163) -> ("ParamDesc"=w1162:string[][])
        n563 = Variant To Data(Variant=w1165, type=0) -> (data=w1160:i32)  [unwired: 1 in, 1 out]
        n564 = local read "Parameter Type"() -> (w1161:i32)
        n565 = Add(x=w1160, y=2) -> (x+y=w1158:i32)
        n566 = Index Array(array=w1162, index (row)=w1161, index (col)=w1158) -> (element=w1159:string)
        n567 = property on="Parameter Check" class="Tbl (strict)"("TipStrip"=w1159) -> ()  [unwired: 2 in, 2 out]
      }
      frame "Next Parameter" {
        n568 = property on="Parameter Check" class="Tbl (strict)"() -> ("EditPos"=w1177:T6, "Value"=w1174:string[][])  [unwired: 2 in, 2 out]
        n569 = Array Size(array=w1174) -> (size(s)=w1173:i32[])
        n570 = call "NextState.vi"("State"="Update Tool Tip", "Queue In"=w1167) -> ()  [unwired: 8 in, 2 out]
        n571 = Index Array(array=w1173) -> (element=w1172:i32)  [unwired: 1 in]
        n572 = Unbundle By Name(w1177) -> ("Row"=w1176:i32)
        n573 = Increment(x=w1176) -> (x+1=w1170:i32)
        n574 = Equal?(x=w1170, y=w1172) -> (x = y?=w1171:bool)
        n575 = Select(t=0, s=w1171, f=w1170) -> (s? t:f=w1168:i32)
        n576 = Bundle By Name(cluster=w1177, "Row"=w1168) -> (w1175:T6)
        n577 = property on="Parameter Check" class="Tbl (strict)"("EditPos"=w1175) -> ()  [unwired: 2 in, 2 out]
      }
      frame "--- Telemetry ---" {
      }
      frame "Read Continuous" {
        # "To send data continously to a subPanel, have queue message sent to main GUI to this state"
        n578 = Unbundle By Name(w1186) -> ("Logger"=w1181:bool, "DebugLogger"=w1180:refnum<queue>, "SubPanelQueue"=w1184:refnum<queue>, "COM Port"=w1187:refnum<visa-resource-name>, "Connected"=w1182:bool)
        n579 = case shown="True" w1182 {
          tunnel: w1187 -> [_ w1203]
          tunnel: w1186 -> [w1188 w1202]
          tunnel: [w1188 w1199] -> w1185
          tunnel: w1184 -> [_ w1195]
          tunnel: w1183 -> [_ w1193]
          tunnel: w1181 -> [_ w1192]
          tunnel: w1180 -> [_ w1191]
          frame False {
          }
          frame True {
            n580 = VISA Read(VISA resource name=w1203, byte count=u32 1024) -> (read buffer=w1189:string, error out=w1201:errorcluster)  [unwired: 1 in, 2 out]
            n581 = Bundle By Name(cluster=w1202, "Error"=w1201) -> (w1199:T2)
            n582 = call "NextState.vi"("State"="Read Continuous", "Queue In"=w1193) -> ()  [unwired: 8 in, 2 out]
            n583 = call "RemoveTrailingComma.vi"("Input String"=w1189) -> ("Output String"=w1190:string)  [unwired: 8 in]
            n584 = Spreadsheet String To Array(delimiter (Tab)=",", format string="%s", spreadsheet string=w1190) -> (array=w1196:dbl[][])  [unwired: 1 in]
            n585 = call "NextState.vi"("Data"=w1196, "State"="Update", "Queue In"=w1195) -> ()  [unwired: 7 in, 2 out]
            n586 = case shown="True" w1192 {
              tunnel: w1191 -> [_ w1207]
              tunnel: w1189 -> [_ w1206]
              frame False {
              }
              frame True {
                n587 = call "NextState.vi"("Data"=w1206, "State"="Read", "Queue In"=w1207) -> ()  [unwired: 7 in, 2 out]
              }
            }
          }
        }
      }
      frame "Read Continuous Binary" {
        # "To send data continously to a subPanel, have queue message sent to main GUI to this state"
        n588 = Unbundle By Name(w1214) -> ("Logger"=w1209:bool, "DebugLogger"=w1208:refnum<queue>, "SubPanelQueue"=w1212:refnum<queue>, "COM Port"=w1215:refnum<visa-resource-name>, "Connected"=w1210:bool)
        n589 = case shown="True" w1210 {
          tunnel: w1215 -> [_ w1228]
          tunnel: w1214 -> [w1216 w1227]
          tunnel: [w1216 w1224] -> w1213
          tunnel: w1212 -> [_ w1223]
          tunnel: w1211 -> [_ w1221]
          tunnel: w1209 -> [_ w1219]
          tunnel: w1208 -> [_ w1218]
          frame False {
          }
          frame True {
            n590 = VISA Read(VISA resource name=w1228, byte count=u32 1024) -> (read buffer=w1217:string, error out=w1226:errorcluster)  [unwired: 1 in, 2 out]
            n591 = String To Byte Array(string=w1217) -> (unsigned byte array=w1220:u8[])
            n592 = Bundle By Name(cluster=w1227, "Error"=w1226) -> (w1224:T2)
            n593 = call "NextState.vi"("State"="Read Continuous Binary", "Queue In"=w1221) -> ()  [unwired: 8 in, 2 out]
            n594 = call "NextState.vi"("Data"=w1220, "State"="Update", "Queue In"=w1223) -> ()  [unwired: 7 in, 2 out]
            n595 = case shown="True" w1219 {
              tunnel: w1218 -> [_ w1232]
              tunnel: w1217 -> [_ w1230]
              frame False {
              }
              frame True {
                n596 = call "NextState.vi"("Data"=w1230, "State"="Read", "Queue In"=w1232) -> ()  [unwired: 7 in, 2 out]
              }
            }
          }
        }
      }
      frame "Read Once" {
        n597 = Unbundle By Name(w1238) -> ("Logger"=w1234:bool, "DebugLogger"=w1233:refnum<queue>, "SubPanelQueue"=w1236:refnum<queue>, "COM Port"=w1239:refnum<visa-resource-name>, "Connected"=w1235:bool)
        n598 = case shown="True" w1235 {
          tunnel: w1239 -> [_ w1253]
          tunnel: w1238 -> [w1240 w1252]
          tunnel: [w1240 w1249] -> w1237
          tunnel: w1236 -> [_ w1245]
          tunnel: w1234 -> [_ w1244]
          tunnel: w1233 -> [_ w1243]
          frame False {
          }
          frame True {
            n599 = VISA Read(VISA resource name=w1253, byte count=u32 1024) -> (read buffer=w1241:string, error out=w1251:errorcluster)  [unwired: 1 in, 2 out]
            n600 = Bundle By Name(cluster=w1252, "Error"=w1251) -> (w1249:T2)
            n601 = call "RemoveTrailingComma.vi"("Input String"=w1241) -> ("Output String"=w1242:string)  [unwired: 8 in]
            n602 = Spreadsheet String To Array(delimiter (Tab)=",", format string="%s", spreadsheet string=w1242) -> (array=w1246:dbl[][])  [unwired: 1 in]
            n603 = call "NextState.vi"("Data"=w1246, "State"="Update", "Queue In"=w1245) -> ()  [unwired: 7 in, 2 out]
            n604 = case shown="True" w1244 {
              tunnel: w1243 -> [_ w1257]
              tunnel: w1241 -> [_ w1256]
              frame False {
              }
              frame True {
                n605 = call "NextState.vi"("Data"=w1256, "State"="Read", "Queue In"=w1257) -> ()  [unwired: 7 in, 2 out]
              }
            }
          }
        }
      }
      frame "Read Integers Once" {
        n606 = Unbundle By Name(w1263) -> ("Logger"=w1258:bool, "DebugLogger"=w1259:refnum<queue>, "SubPanelQueue"=w1261:refnum<queue>, "COM Port"=w1264:refnum<visa-resource-name>, "Connected"=w1260:bool)
        n607 = case shown="True" w1260 {
          tunnel: w1264 -> [_ w1279]
          tunnel: w1263 -> [w1265 w1278]
          tunnel: [w1265 w1275] -> w1262
          tunnel: w1261 -> [_ w1271]
          tunnel: w1259 -> [_ w1269]
          tunnel: w1258 -> [_ w1268]
          frame False {
          }
          frame True {
            n608 = VISA Read(VISA resource name=w1279, byte count=u32 1024) -> (read buffer=w1266:string, error out=w1277:errorcluster)  [unwired: 1 in, 2 out]
            n609 = Bundle By Name(cluster=w1278, "Error"=w1277) -> (w1275:T2)
            n610 = call "RemoveTrailingComma.vi"("Input String"=w1266) -> ("Output String"=w1267:string)  [unwired: 8 in]
            n611 = Spreadsheet String To Array(delimiter (Tab)=",", format string="%s", spreadsheet string=w1267, array type (2D Dbl)=0) -> (array=w1272:i32[][])
            n612 = call "NextState.vi"("Data"=w1272, "State"="Update", "Queue In"=w1271) -> ()  [unwired: 7 in, 2 out]
            n613 = case shown="False" w1268 {
              tunnel: w1269 -> [_ w1283]
              tunnel: w1266 -> [_ w1282]
              frame False {
              }
              frame True {
                n614 = call "NextState.vi"("Data"=w1282, "State"="Read", "Queue In"=w1283) -> ()  [unwired: 7 in, 2 out]
              }
            }
          }
        }
      }
      frame "Read Integers Continuous" {
        n615 = Unbundle By Name(w1290) -> ("Logger"=w1285:bool, "DebugLogger"=w1286:refnum<queue>, "SubPanelQueue"=w1288:refnum<queue>, "COM Port"=w1291:refnum<visa-resource-name>, "Connected"=w1287:bool)
        n616 = case shown="True" w1287 {
          tunnel: w1291 -> [_ w1308]
          tunnel: w1290 -> [w1292 w1307]
          tunnel: [w1292 w1304] -> w1289
          tunnel: w1288 -> [_ w1300]
          tunnel: w1286 -> [_ w1298]
          tunnel: w1285 -> [_ w1297]
          tunnel: w1284 -> [_ w1293]
          frame False {
          }
          frame True {
            n617 = VISA Read(VISA resource name=w1308, byte count=u32 1024) -> (read buffer=w1295:string, error out=w1306:errorcluster)  [unwired: 1 in, 2 out]
            n618 = Bundle By Name(cluster=w1307, "Error"=w1306) -> (w1304:T2)
            n619 = call "NextState.vi"("State"="Read Integers Continuous", "Queue In"=w1293) -> ()  [unwired: 8 in, 2 out]